vi "UHR-Fleezers Control (host) - 12.7c.vi"() -> ()   [LabVIEW 2012] (continued)
  T19 = typedef "nirio_resource_hc.ctl" = tag
  T20 = typedef "openfpgaref.8.6.ctl" = refnum<k20>
  T21 = enum16{"empty", "write", "read oldest (queue)", "read newest (stack)", "read all"}
  T22 = cluster{"New Image":T2, "New Image":T2, "New Image":T2, "New Image":T2, "New Image":T2}
  T23 = typedef "XDNodeRunTimeDep.lvlib/timing_clust.ctl" = cluster{"Expected End [f-1]":u64, "Actual End [f-1]":u64, "Finished Late? [f-1]":bool, "Expected End [i-1]":u64, "Actual End [i-1]":u64, "Finished Late? [i-1]":bool, "Expected Start [i]":u64, "Actual Start [i]":u64, "Expected Start [f]":u64, "Actual Start [f]":u64, "Source Name":string, "Structure Name":string, "Period":i64, "Deadline":i64, "Offset":i64, "Start":i64, "Priority":i32, "Timeout":i32, "Mode":T24, "Wakeup Reason":T25, "Error":errorcluster, "Source Type":string, "Secondary Source Type":string, "Global End Time":u64, "Global Start Time":u64, "Frame Duration":u64, "Iteration Duration":u64, "Assigned CPU":i32, "I/O Scan Engine Mode":u32}
  T24 = typedef "XDNodeRunTimeDep.lvlib/nitl_modes.ctl" = enum32{"No Change", "Process missed periods, maintain original phase", "Discard missed periods, maintain original phase", "Process missed periods, ignore original phase", "Discard missed periods, ignore original phase"}
  T25 = typedef "XDNodeRunTimeDep.lvlib/wakeup.ctl" = enum32{"Normal", "Aborted", "Asynchronous wakeup", "Timing source error", "Timed loop error", "Timeout"}
  T26 = enum16{"big-endian, network order", "native, host order", "little-endian"}
  T27 = enum16{"open", "replace", "create", "open or create", "replace or create", "replace or create with confirmation"}
  T28 = cluster{"Scan Range AOD (nm) 2":dbl, "Step Size AOD (nm) 2":dbl, "Scan Speed AOD (nm/s) 2":dbl, "Number of scans (AOD) 2":u16, "Label":string}
  T29 = cluster{"[0]":dbl, "[1]":dbl, "[2]":dbl, "[3]":dbl, "[4]":dbl, "[5]":dbl}
  T30 = cluster{"Diameter (mm)":dbl, "Units":dbl, "Volume":dbl, "Rate":dbl}
  T31 = cluster{"Left":i32, "Top":i32, "Width":u32, "Height":u32}
  T32 = cluster{cluster{"Left":i32, "Top":i32, "Width":u32, "Height":u32}}[]
  T33 = enum32{"Status", "Sample Stage", "Syringe Pump", "Trap Control (RF)", "APD Counting", "Fluorescence Laser Control", "Trap AI", "Video", "FPGA"}
  T34 = enum32{"Status", "Sample Stage", "Syringe Pump", "Trap Control (RF)", "APD Counting", "Fluorescence Laser Control", "Trap AI", "Video", "FPGA", "Misc. Configuration"}
  T35 = enum32{"setting", "request", "request control", "info", "statistics", "system settings", "I/O sub system", "HRT control", "camera descriptions", "device specific data", "event sub system settings", "event sub system results", "image memory manager"}
  T36 = typedef "AviRefnum.ctl" = refnum<k1>
  T37 = typedef "imagedata.ctl" = cluster{"image type":i32, "image depth":i32, "image":u8[], "mask":u8[], "colors":u32[], "Rectangle":cluster{"left":i16, "top":i16, "right":i16, "bottom":i16}}
  T38 = enum32{"Normal Display", "Dual Display (APD)", "FFT", "High Res Display"}
  T39 = cluster{"Origin Pixel":cluster{"X":sgl, "Y":sgl}, "Angle Relative to Horizontal (deg)":sgl, "Axis Reference":u32}
  T40 = typedef "Simple Grid Descriptor" = cluster{"X Step":sgl, "Y Step":sgl, "Unit":T41}
  T41 = typedef "Image Unit" = enum32{"Undefined", "Angström", "Micrometer", "Millimeter", "Centimeter", "Meter", "Kilometer", "Microinch", "Inch", "Feet", "Nautical miles", "Standard miles", "Steps"}
  T42 = cluster{"averaging mode":u16, "weighting mode":u16, "number of averages":u32}
  T43 = cluster{"dB On (F)":bool, "unwrap phase (F)":bool, "convert to degree (F)":bool}
  T44 = cluster{string, string, string, string, string, string, string, string}
  T45 = cluster{string, string, string, string, string, string, string, string, string, string, string, string}
  T46 = cluster{string, string, string, string, string, string, string, string, string, string, string, string, string}
  T47 = cluster{string, string, string, string, string, string, string, string, string, string, string, string, string, string}
  T48 = cluster{"BD 1 Frequency 1 (MHz)":dbl, "BD 1 Frequency 2 (MHz)":dbl}
  T49 = cluster{"f0":dbl, "df":dbl, "magnitude":dbl[]}[][]
  T50 = cluster{"Comment (data description)":string, "Channel 1 Buffer":string, "Channel 2 Buffer":string, "Channel 3 Buffer":string, "Title":string, "DNA Construct":string, "Bead diameter":dbl, "Name":string}
diagram:
  w14 = u16 10 items=["1.0"=10, "1.5"=15, "2.0"=20] ("stop bits (10: 1 bit)")
  w80 = u16 20 items=["1.0"=10, "1.5"=15, "2.0"=20] ("stop bits (10: 1 bit)")
  w83 = u16 20 items=["1.0"=10, "1.5"=15, "2.0"=20] ("stop bits (10: 1 bit)")
  w109 = u16 20 items=["1.0"=10, "1.5"=15, "2.0"=20] ("stop bits (10: 1 bit)")
  w20 = T18 2 items=["Grayscale (U8)", "Grayscale (I16)", "Grayscale (SGL)", "Complex (CSG)", "RGB (U32)", "HSL (U32)", "RGB (U64)", "Grayscale (U16)"] ("Image Type")
  w239 = 10.0 ("y")
  w238 = 32767.0 ("y")
  w254 = 6.0  # clock mult.
  w255 = 49152000.0  # TCXO frequ.
  # "Trap X limits"
  # "What are these?"
  # "I don't think you need to do this.\nEverytime you want to adjust phase you always set this anyway.\nSince we removed the separate +/- controls.\n\nHaven't added for added fl lasers.  Should remove this code."
  # "Bottom 1 Harvard"
  # "Top 3 Harvard"
  # "Center Harvard"
  # "Bottom 1 Harvard"
  # "Top 3 Harvard"
  # "Center Harvard"
  n1 = Build Array("DIO count 1 (ticks)", "DIO count 2 (ticks)", "DIO count 3 (ticks)") -> (w160:u16[])
  n2 = xnode "Open FPGA VI Reference"("resource name"=T19 "750kHzDAQ") -> ("FPGA VI Reference Out"=w263:T20, "error out"=w262:errorcluster)  [unwired: 1 in]
  n3 = local read "AO1"() -> (w233:dbl)
  n4 = local read "AO2"() -> (w232:dbl)
  n5 = local read "Scan Increment (MHz)"() -> (w250:dbl)
  n6 = local read "Continuous MCL Scanning"() -> (w220:bool)
  n7 = local read "Fast Scan Dir"() -> (w219:bool)
  n8 = xnode "Invoke Method"("FPGA VI Reference In"=w263, "error in"=w262) -> ("FPGA VI Reference Out"=w1:T20, "error out"=w179:errorcluster)
  n9 = local read "Number of scans (MCL)"() -> (w221:u64)
  n10 = Multiply(x=w233, y=w238) -> (x*y=w235:dbl)
  n11 = Multiply(x=w232, y=w238) -> (x*y=w237:dbl)
  n12 = Divide(x=w235, y=w239) -> (x/y=w234:dbl)
  n13 = Divide(x=w237, y=w239) -> (x/y=w236:dbl)
  n14 = To Word Integer(number=w234) -> (16bit integer=w231:i16)
  n15 = To Word Integer(number=w236) -> (16bit integer=w230:i16)
  n16 = Not(x=w219) -> (.not. x?=w214:bool)
  n17 = local read "Cycles/step (MCL)"() -> (w222:u64)
  n18 = Multiply(x=w250, y=1000.0) -> (x*y=w257:dbl)
  n19 = local read "Scan steps (MCL)"() -> (w223:u64)
  n20 = local read "Desired Scan Incr (V)"() -> (w225:dbl)
  n21 = Scale By Power Of 2(n=48, x=w257) -> (x*2^n=w258:dbl)
  n22 = Unbundle By Name(cluster{"output high":i16, "output low":i16} {"output high"=3000, "output low"=0} ("FB output range 1")) -> ("output high"=w61:i16, "output low"=w60:i16)
  n23 = Multiply(x=w255, y=w254) -> (x*y=w253:dbl)
  n24 = Divide(x=w258, y=w253) -> (x/y=w252:dbl)
  n25 = local read "Setpoints (V)"() -> (w269:cluster{"Set 1":dbl, "Set 2":dbl})
  n26 = To Quad Integer(1:w252) -> (0:w249:i64)
  n27 = Divide(x=40000000.0, y="AI Count (ticks)") -> (x/y=w210:dbl)
  n28 = Multiply(x=w225, y=32767.0) -> (x*y=w227:dbl)
  n29 = local read "Trap Intensity PID Gains"() -> (w264:T9)
  n30 = local read "Next trap write delay (ticks)"() -> (w6:u8)
  n31 = local read "XY phase ext loop method"() -> (w5:bool)
  n32 = local read "Amp switch delay 2"() -> (w4:u8)
  n33 = local read "BD 2 Delay (Ticks) 2"() -> (w3:u8)
  n34 = local read "BD 1 Delay (ticks) 2"() -> (w2:u8)
  n35 = local write "Trap Pos FIFO Timeout"(u16 0 ("Trap Pos FIFO Timeout")) -> ()
  n36 = local read "Number Interlace Sets"() -> (w153:u8)
  n37 = Split 1D Array(array=w160, index=w153) -> (first subarray=w162:u16[])  [unwired: 1 out]
  n38 = Add Array Elements(numeric array=w162) -> (sum=w161:u16)
  n39 = local read "# Samples/channel"() -> (w242:u32)
  n40 = local read "Number of F/B Scans (AOD)"() -> (w243:u16)
  n41 = local read "Not-Interlacing Set"() -> (w152:enum32{"Set 1", "Set 2", "Set 3"})
  n42 = To Unsigned Byte Integer(number=w152) -> (unsigned 8bit integer=w158:u8)
  n43 = Index Array(array=w160, index=w158) -> (element=w159:u16)
  n44 = local read "Feedback On/Off"() -> (w272:cluster{"Set 1":bool, "Set 2":bool})
  n45 = local read "BD 2 Delay (Ticks)"() -> (w7:u8)
  n46 = local read "BD 1 Delay (ticks)"() -> (w8:u8)
  n47 = local read "Scan steps (AOD)"() -> (w248:u64)
  n48 = local read "All FB On/Off"() -> (w273:bool)
  n49 = local read "Cycles/step (AOD)"() -> (w247:u64)
  n50 = local write "AI rate (Hz)"(w210) -> ()
  n51 = Divide(x=w227, y=10.0) -> (x/y=w226:dbl)
  n52 = Multiply(x=w248, y=w247) -> (x*y=w246:u64)
  n53 = Unbundle By Name(w264) -> ("proportional gain (Kc)"=w65:i16, "integral gain (Kc*Ts/Ti)"=w64:i16, "derivative gain (Kc*Td/Ts)"=w63:i16)
  n54 = property on="AI Count (ticks)" class="DigNum (strict)"("Val(Sgnl)"="AI Count (ticks)") -> ()  [unwired: 2 in, 2 out]
  n55 = Multiply(x=3276.7, y=w269) -> (x*y=w268:cluster{"Set 1":dbl, "Set 2":dbl})
  n56 = To Word Integer(number=w226) -> (16bit integer=w224:i16)
  n57 = Multiply(x=w246, y=u64 2) -> (x*y=w244:u64)
  n58 = Divide(x=w210, y="FPGA Ave.") -> (x/y=w211:dbl)
  n59 = To Word Integer(number=w268) -> (16bit integer=w267:cluster{"Set 1":i16, "Set 2":i16})
  n60 = Multiply(x=w244, y=w243) -> (x*y=w241:u64)
  n61 = local read "Sets to FIFO (Traps)"() -> (w69:T15)
  n62 = local write "Ave. Rate (Hz)"(w211) -> ()
  n63 = Divide(x=w241, y=w242) -> (x/y=w240:dbl)
  n64 = Unbundle By Name(w267) -> ("Set 1"=w266:i16, "Set 2"=w265:i16)
  n65 = local read "2D or 1D Scan"() -> (w171:bool)
  n66 = local write "Data points/scans"(w241) -> ()
  n67 = local read "Scan BD"() -> (w259:bool)
  n68 = And(x=w272, y=w273) -> (x .and. y?=w271:cluster{"Set 1":bool, "Set 2":bool})
  n69 = local write "Data points/scan (f/b)"(w244) -> ()
  n70 = Reciprocal(x=w211) -> (1/x=w212:dbl)
  n71 = local read "N Acq Sets (Traps + Fl.)"() -> (w203:i16)
  n72 = local write "N sets should be saved"(w240) -> ()
  n73 = Unbundle By Name(w271) -> ("Set 1"=w275:bool, "Set 2"=w274:bool)
  n74 = local read "Interlace"() -> (w154:bool)
  n75 = Select(t=w161, s=w154, f=w159) -> (s? t:f=w151:u16)
  n76 = local write "Update Count (MCL)"(w151) -> ()
  n77 = local write "Total Counts (ticks)"(w151) -> ()
  n78 = local write "Ave. Period (s)"(w212) -> ()
  n79 = Unbundle By Name(w69) -> ("Set 1"=w68:bool, "Set 2"=w67:bool, "Set 3"=w66:bool)
  n80 = property on="2D or 1D Scan" class="Bool (strict)"("Val(Sgnl)"=w171) -> ()  [unwired: 2 in, 2 out]
  n81 = xnode "Read/Write Control"("FPGA VI Reference In"=w170, "error in"=w179, "ai count"="AI Count (ticks)", "Interlace ON/OFF"=w154, "Number Interlace Cycles"=w153, "Set 1"=w68, "Set 2"=w67, "Set 3"=w66, "FB On/Off Set 1"=w275, "FB On/Off Set 2"=w274, "Interlace Off Parameters"=w152, "FB Setpoint Set 1"=w266, "FB Setpoint Set 2"=w265, "P1"=w65, "I1"=w64, "D1"=w63, "FB1 output high"=w61, "FB1 output low"=w60, "Cycles per step"=w247, "Scan BD"=w259, "Number of scans"=w243, "Scan steps"=w248, "Scan freq.  increment"=w249, "AO1"=w231, "AO2"=w230, "Scan freq.  increment (MCL)"=w224, "Scan steps (MCL)"=w223, "Cycles per step (MCL)"=w222, "Number of scans (MCL)"=w221, "MCL count"=w151, "Cont. Scan (MCL)"=w220, "MCL Scan Axis"=w214, "1D or 2D Scan?"=w171, "N of AI1 Int Acq Sets"=w203, "Amp switch delay"="Amp switch delay", "Swap F1 and F2"="Swap F1 and F2", "APD to FIFO"=FALSE, "DIO count 1 (ticks)"="DIO count 1 (ticks)", "DIO count 2 (ticks)"="DIO count 2 (ticks)", "DIO count 3 (ticks)"="DIO count 3 (ticks)", "BD 1 Delay (ticks)"=w8, "BD 2 Delay (Ticks)"=w7, "Next trap write delay (ticks)"=w6, "XY phase ext loop method"=w5, "Amp switch delay 2"=w4, "BD 2 Delay (Ticks) 2"=w3, "BD 1 Delay (ticks) 2"=w2) -> ("FPGA VI Reference Out"=w25:T20, "error out"=w24:errorcluster)  [unwired: 1 in]
  n82 = local read "Laser interlacing mode"() -> (w150:enum32{"Laser ON", "Laser OFF", "Interlace"})
  n83 = local read "Green Laser ON"() -> (w149:bool)
  n84 = local read "Trap Pos. FB Range"() -> (w59:T12)
  n85 = local read "Trap Pos. FB Gains"() -> (w58:T11)
  n86 = Multiply(x="Green Intensity % (FB OFF)", y=655.35) -> (x*y=w142:dbl)
  n87 = local read "Invert laser interlacing"() -> (w38:bool)
  n88 = local read "Trap Pos. AI1 X Pre-scale"() -> (w97:u16)
  n89 = Multiply(x="Green FB Setpoint (mV)", y=3.2767) -> (x*y=w139:dbl)
  n90 = local read "Trap Pos FB Int Count"() -> (w91:u16)
  n91 = local read "Differential FB?"() -> (w85:bool)
  n92 = local read "Neg. TTrig FPGA"() -> (w87:bool)
  n93 = Multiply(x="Red FB Setpoint (mV)", y=3.2767) -> (x*y=w46:dbl)
  n94 = To Unsigned Word Integer(number=w142) -> (unsigned 16bit integer=w140:u16)
  n95 = Multiply(x="Red Intensity % (FB OFF)", y=655.35) -> (x*y=w42:dbl)
  n96 = To Word Integer(number=w139) -> (16bit integer=w137:i16)
  n97 = Unbundle By Name("Green FB Gains") -> ("proportional gain (Kc)"=w50:i16, "integral gain (Kc*Ts/Ti)"=w49:i16, "derivative gain (Kc*Td/Ts)"=w48:i16)
  n98 = Unbundle By Name("Red FB Gains") -> ("proportional gain (Kc)"=w35:i16, "integral gain (Kc*Ts/Ti)"=w34:i16, "derivative gain (Kc*Td/Ts)"=w33:i16)
  n99 = case shown="False" w149 {
    tunnel: w150 -> [_ w301]
    tunnel: [enum32{"Laser ON", "Laser OFF", "Interlace"}."Laser OFF" ("Green laser mode") w301] -> w37
    frame False {
    }
    frame True {
    }
  }
  n100 = To Word Integer(number=w46) -> (16bit integer=w43:i16)
  n101 = Unbundle By Name(w58) -> ("proportional gain (Kc)"=w54:fxp<+/-,16,8>, "integral gain (Kc*Ts/Ti)"=w53:fxp<+/-,16,8>, "derivative gain (Kc*Td/Ts)"=w52:fxp<+/-,16,8>)
  n102 = To Unsigned Word Integer(number=w42) -> (unsigned 16bit integer=w39:u16)
  n103 = Unbundle By Name(w59) -> ("output high"=w57:fxp<+/-,16,1>, "output low"=w55:fxp<+/-,16,1>)
  n104 = local read "Trap Pos FB Monitor\nT1 or T2"() -> (w102:bool)
  n105 = local read "Trap Pos FB Negate Action"() -> (w101:bool)
  n106 = local read "Trap Pos. FB Offset Factor"() -> (w100:i64)
  n107 = local read "Trap Pos. FB Mult Factor"() -> (w99:i64)
  n108 = xnode "Read/Write Control"("FPGA VI Reference In"=w25, "error in"=w24, "Invert GI 2"=w38, "Operating Mode 2"=w37, "P3"=w50, "I3"=w49, "D3"=w48, "Green FB Setpoint"=w137, "Green FB On/Off"="Green FB On/Off", "Current Out"=w140, "Green int current ON count adj"="Green int current ON count adj", "Operating Mode"=w37, "Invert GI"=w38, "Trap Pos FB Monitor T1 or T2"=w102, "Trap Pos FB Negate Action"=w101, "Trap Pos. FB Offset Factor"=w100, "Trap Pos. FB Mult Factor"=w99, "Force feedback"=FALSE, "AI1 X Scale"=w97, "Trap Pos to FIFO"=TRUE, "Trap Pos FB Int Count"=w91, "TTrig Negate Pos"=w87, "FB Trig Integrate"="FB Trig Integrate", "Diff FB Measurement?"=w85, "Negate Diff?"="Negate Diff?", "P2"=w54, "I2"=w53, "D2"=w52, "FB2 output high"=w57, "FB2 output low"=w55, "Red FB Setpoint"=w43, "RI Current Out"=w39, "Red Laser Operating Mode"=w37, "RI Operating Mode 2"=w37, "Invert RI 2"=w38, "Invert RI"=w38, "P4"=w35, "I4"=w34, "D4"=w33, "Red FB On/Off"="Red FB On/Off") -> ("FPGA VI Reference Out"=w29:T20, "error out"=w31:errorcluster)
  n109 = stacked-sequence {
    tunnel: w31 -> [_ _ _ w312]
    tunnel: [_ _ _ w312] -> w30
    tunnel: w29 -> [_ _ _ w313]
    tunnel: [_ _ _ w313] -> w28
    frame #0 {
      w302 = T21."empty" ("mode")
      # "Clear external fluorescence triggering FIFO"
      # "APD loop counts"
      # "Fluorescence loop counts (rates)"
      n110 = local read "APD Integration Time (s)"() -> (w304:dbl)
      n111 = local read "Interlace ON count"() -> (w305:u16)
      n112 = call "Smart Buffer (DBL) 1.vi"("mode"=w302) -> ()  [unwired: 5 in, 6 out]
      n113 = call "Smart Buffer (DBL) 2.vi"("mode"=w302) -> ()  [unwired: 5 in, 6 out]
      n114 = property on="APD Integration Time (s)" class="DigNum (strict)"("Val(Sgnl)"=w304) -> ()  [unwired: 2 in, 2 out]
      n115 = property on="Interlace ON count" class="DigNum (strict)"("Val(Sgnl)"=w305) -> ()  [unwired: 2 in, 2 out]
      "Number of APDs" <- 3.0 ("Number of APDs")
    }
    frame #1 {
      # "Number of APDs affects\nAPD DMA transfer"
      # "General settings for all lasers:"
      # "And includes all laser\nON/OFF settings"
      # "Fluorescent lasers settings:"
      # "Blue laser settings:"
      n116 = local read "Laser interlacing mode"() -> (w307:enum32{"Laser ON", "Laser OFF", "Interlace"})
      n117 = local read "Invert laser interlacing"() -> (w306:bool)
      n118 = local read "Blue FB On/Off"() -> (w308:bool)
      n119 = property on="Blue FB On/Off" class="Bool (strict)"("Val(Sgnl)"=w308) -> ()  [unwired: 2 in, 2 out]
      n120 = property on="Invert laser interlacing" class="Bool (strict)"("Val(Sgnl)"=w306) -> ()  [unwired: 2 in, 2 out]
      n121 = property on="Laser interlacing mode" class="RadioBtnsControl (strict)"("Val(Sgnl)"=w307) -> ()  [unwired: 2 in, 2 out]
    }
    frame #2 {
      w309 = path "C:/Home/wheeler/Comstock-LabView-Link.udl" ("connection information")
      # "Initialize the database connection"
      n122 = call-poly <vilib>:"DB Tools Open Connection.vi"("connection information"=w309) -> ("connection reference"=w310:T17)  [unwired: 7 in, 1 out]
      "connection reference" <- w310
      n123 = local write "connection reference"(w310) -> ()
      n124 = local write "Database link"(w309) -> ()
    }
    frame #3 {
      n125 = Wait (ms)(milliseconds to wait=u32 1000) -> ()  [unwired: 1 out]
    }
  }
  n126 = local write "Offset (nm)"(0.0 ("Offset (nm)")) -> ()
  n127 = local write "Bead Mean (nm)"(0.0 ("Bead Mean (nm)")) -> ()
  n128 = case shown="\"2axisAOD\"" "1axis AOM vs 2 axis AOD" {
    tunnel: [T16 {"Minimum"=0.0, "Maximum"=40.0, "Increment"=0.1} ("Min Max Inc") T16 {"Minimum"=60.0, "Maximum"=90.0, "Increment"=1.0} ("Min Max Inc")] -> w11
    tunnel: [T16 {"Minimum"=0.0, "Maximum"=45.0, "Increment"=1.0} ("Data Entry Limits") T16 {"Minimum"=0.0, "Maximum"=50.0, "Increment"=1.0} ("Data Entry Limits")] -> w9
    frame "2axisAOD" {
      # "Amp Limits"
      # "Freq Limits"
      n129 = disable-structure shown="Disabled" {
        frame Disabled {
          w319 = 35.0 ("BD 1 Amplitude 1 (%)")
          w320 = 30.0 ("BD 1 Frequency 1 (MHz)")
          n130 = local write "BD 1 Frequency 1 (MHz)"(w320) -> ()
          n131 = local write "BD 1 Frequency 2 (MHz)"(w320) -> ()
          n132 = local write "BD 1 Amplitude 2 (%)"(w319) -> ()
          n133 = local write "BD 1 Amplitude 1 (%)"(w319) -> ()
          n134 = local write "BD 2 Frequency 1 (MHz)"(w320) -> ()
          n135 = local write "BD 2 Amplitude 1 (%)"(w319) -> ()
          n136 = local write "BD 2 Frequency 2 (MHz)"(w320) -> ()
          n137 = local write "BD 2 Amplitude 2 (%)"(w319) -> ()
        }
        frame Enabled {
        }
      }
      n138 = local write "BD 2 Delay (Ticks)"(u8 47 ("BD 2 Delay (Ticks)")) -> ()
      n139 = local write "All FB On/Off"(FALSE ("All FB On/Off")) -> ()
      n140 = local write "Number Interlace Sets"(u8 2 ("Number Interlace Sets")) -> ()
    }
    frame "1axis", Default {
      # "Amp Lmits"
      # "Freq Limits"
    }
  }
  n141 = xnode "Invoke Method"("FPGA VI Reference In"=w28, "error in"=w30, "Requested Depth"="Trap AI FIFO Depth") -> ("FPGA VI Reference Out"=w105:T20, "error out"=w104:errorcluster)  [unwired: 1 out]
  n142 = xnode "Invoke Method"("FPGA VI Reference In"=w105, "error in"=w104, "Requested Depth"="Trap Position FIFO Depth") -> ("FPGA VI Reference Out"=w93:T20, "error out"=w92:errorcluster)  [unwired: 1 out]
  n143 = flat-sequence "Safety limits on RF frequencies and amplitudes (for AOM protection)" {
    tunnel: w1 -> [w327]
    tunnel: [w327] -> w170
    tunnel: [w324] -> w169
    tunnel: [w323] -> w168
    tunnel: [w325] -> w166
    tunnel: [w326] -> w167
    tunnel: w11 -> [w324]
    tunnel: w9 -> [w323]
    frame #0 {
      w326 = T16 {"Minimum"=0.0, "Maximum"=40.0, "Increment"=0.1} ("Min Max Inc")
      w325 = T16 {"Minimum"=0.0, "Maximum"=45.0, "Increment"=1.0} ("Data Entry Limits")
      n144 = property on="BD 2 Frequency 1 (MHz)" class="DigNum (strict)"("Data Range"=w326) -> ()  [unwired: 2 in, 2 out]
      n145 = property on="BD 2 Frequency 3 (MHz)" class="DigNum (strict)"("Data Range"=w326) -> ()  [unwired: 2 in, 2 out]
      n146 = property on="BD 2 Frequency 2 (MHz)" class="DigNum (strict)"("Data Range"=w326) -> ()  [unwired: 2 in, 2 out]
      n147 = property on="BD 1 Frequency 1 (MHz)" class="DigNum (strict)"("Data Range"=w324) -> ()  [unwired: 2 in, 2 out]
      n148 = property on="BD 1 Frequency 2 (MHz)" class="DigNum (strict)"("Data Range"=w324) -> ()  [unwired: 2 in, 2 out]
      n149 = property on="BD 1 Frequency 3 (MHz)" class="DigNum (strict)"("Data Range"=w324) -> ()  [unwired: 2 in, 2 out]
      n150 = property on="BD 2 Amplitude 1 (%)" class="DigNum (strict)"("Data Range"=w325) -> ()  [unwired: 2 in, 2 out]
      n151 = property on="BD 2 Amplitude 2 (%)" class="DigNum (strict)"("Data Range"=w325) -> ()  [unwired: 2 in, 2 out]
      n152 = property on="BD 2 Amplitude 3 (%)" class="DigNum (strict)"("Data Range"=w325) -> ()  [unwired: 2 in, 2 out]
      n153 = property on="BD 1 Amplitude 3 (%)" class="DigNum (strict)"("Data Range"=w323) -> ()  [unwired: 2 in, 2 out]
      n154 = property on="BD 1 Amplitude 2 (%)" class="DigNum (strict)"("Data Range"=w323) -> ()  [unwired: 2 in, 2 out]
      n155 = property on="BD 1 Amplitude 1 (%)" class="DigNum (strict)"("Data Range"=w323) -> ()  [unwired: 2 in, 2 out]
      "X RF Frequency Limits (MHz)" <- w324
      "X RF Amplitude Limits (%)" <- w323
      "Y RF Amplitude Limits (%)" <- w325
      "Y RF Frequency Limits (MHz)" <- w326
    }
  }
  n156 = xnode "Invoke Method"("FPGA VI Reference In"=w93, "error in"=w92) -> ("FPGA VI Reference Out"=w178:T20, "error out"=w177:errorcluster)  [unwired: 1 in]
  n157 = flat-sequence "Initial FPGA Loop Relative Phase Adjustment" {
    tunnel: "Initial Phase Adjustment (AI1)" -> [w342]
    tunnel: "Initial Phase Adjustment (GI)" -> [w341]
    tunnel: w178 -> [w340]
    tunnel: w177 -> [w339]
    tunnel: "Initial Phase Adj. (MCL)" -> [w338]
    tunnel: [w343] -> w187
    tunnel: [w337] -> w183
    tunnel: "Initial Phase Adjustment (APD Acq)" -> [w336]
    tunnel: "Initial Phase Adjustment (APD 1 Gate)" -> [w335]
    tunnel: "Initial Phase Adjustment (Green FB)" -> [w334]
    tunnel: "Initial Phase Adjustment (GI) 2" -> [w333]
    tunnel: "Initial Phase Adjustment (APD 2 Gate)" -> [w332]
    tunnel: "Initial Phase Adjustment (RI)" -> [w331]
    tunnel: "Initial Phase Adjustment (BI DO)" -> [w330]
    tunnel: "Initial Phase Adjustment (BI AO)" -> [w329]
    tunnel: "Initial Phase Adjustment (APD 3 Gate)" -> [w328]
    tunnel: w187 -> [w345]
    tunnel: [w346] -> w184
    tunnel: w183 -> [w346]
    tunnel: [w345] -> w182
    tunnel: w184 -> [w349]
    tunnel: w182 -> [w348]
    tunnel: [w351] -> w181
    tunnel: [w350] -> w180
    tunnel: [w353] -> w185
    tunnel: [w354] -> w186
    tunnel: w181 -> [w354]
    tunnel: w180 -> [w353]
    frame #0 {
      n158 = xnode "Read/Write Control"("FPGA VI Reference In"=w340, "error in"=w339, "Phase count adjustment"=w342, "Phase count adjustment (GI)"=w341, "Phase count adjustment (MCL)"=w338, "Phase Count Adjustment (APD Acq)"=w336, "Phase count adjustment (APD 1 Gate)"=w335, "Phase count adjustment (APD 2 Gate)"=w332, "Phase count adjustment (Green FB)"=w334, "Phase count adjustment (GI) 2"=w333, "Phase count adjustment (RI)"=w331, "Phase count adjustment (BI AO)"=w329, "Phase count adjustment (BI D)"=w330, "Phase count adjustment (APD 3 Gate)"=w328) -> ("FPGA VI Reference Out"=w337:T20, "error out"=w343:errorcluster)
    }
    frame #1 {
      n159 = Wait (ms)(milliseconds to wait=u32 100) -> ()  [unwired: 1 out]
    }
    frame #2 {
      w347 = TRUE
      n160 = xnode "Read/Write Control"("FPGA VI Reference In"=w349, "error in"=w348, "+ phase"=w347, "+ phase (GI)"=w347, "+ phase (MCL)"=w347, "+ phase (APD Acq)"=w347, "+ phase (APD 1 Gate)"=w347, "+ phase (APD 2 Gate)"=w347, "+ phase (Green FB)"=w347, "+ phase (GI) 2"=w347, "+ phase (RI)"=w347, "+ phase (BI AO)"=w347, "+ phase (BI D)"=w347, "+ phase (APD 3 Gate)"=w347) -> ("FPGA VI Reference Out"=w350:T20, "error out"=w351:errorcluster)
    }
    frame #3 {
      n161 = Wait (ms)(milliseconds to wait=u32 100) -> ()  [unwired: 1 out]
    }
  }
  n162 = local read "Phase adj. (Green FB)"() -> (w163:i16)
  n163 = local read "Phase adj. (GI) 2"() -> (w143:i16)
  n164 = local read "Phase adjust (MCL)"() -> (w215:i16)
  n165 = local read "Phase adj. (AI1)"() -> (w217:i16)
  n166 = local read "Phase adj. (GI)"() -> (w216:i16)
  n167 = xnode "Read/Write Control"("FPGA VI Reference In"=w185, "error in"=w186, "Phase count adjustment"=w217, "Phase count adjustment (GI)"=w216, "Phase count adjustment (MCL)"=w215, "Phase Count Adjustment (APD Acq)"="Phase Adj. (APD Acq)", "Phase count adjustment (APD 1 Gate)"="Phase Adj. (APD 1 Gate)", "Phase count adjustment (APD 2 Gate)"="Phase Adj. (APD 2 Gate)", "Phase count adjustment (Green FB)"=w163, "Phase count adjustment (GI) 2"=w143) -> ("FPGA VI Reference Out"=w129:T20, "error out"=w192:errorcluster)
  n168 = call "Initialize RF boards - interlace 3.vi"("error in"=w192, "FPGA VI Reference In"=w129) -> ("error out"=w190:errorcluster, "FPGA VI Reference Out"=w191:T20)
  n169 = call "set RF board frequency - interlace.vi"("Board 2 Frequency Limits"=w167, "Board 1 Frequency Limits"=w169, "error in"=w190, "FPGA VI Reference In"=w191, "Board 2 Frequency 3 (MHz)"="BD 2 Frequency 3 (MHz)", "Board 1 Frequency 3 (MHz)"="BD 1 Frequency 3 (MHz)", "Board 2 Frequency 2 (MHz)"="BD 2 Frequency 2 (MHz)", "Board 2 Frequency 1 (MHz)"="BD 2 Frequency 1 (MHz)", "Board 1 Frequency 2 (MHz)"="BD 1 Frequency 2 (MHz)", "Board 1 Frequency 1  (MHz)"="BD 1 Frequency 1 (MHz)") -> ("error out"=w290:errorcluster, "FPGA VI Reference Out"=w291:T20)
  n170 = call "set RF board amplitude - interlace.vi"("Board 2 Amplitude Limits"=w166, "Board 1 Amplitude Limits"=w168, "error in"=w290, "FPGA VI Reference In"=w291, "Board 2 Amplitude 3 (%)"="BD 2 Amplitude 3 (%)", "Board 1 Amplitude 3 (%)"="BD 1 Amplitude 3 (%)", "Board 2 Amplitude 2 (%)"="BD 2 Amplitude 2 (%)", "Board 2 Amplitude 1 (%)"="BD 2 Amplitude 1 (%)", "Board 1 Amplitude 2 (%)"="BD 1 Amplitude 2 (%)", "Board 1 Amplitude 1 (%)"="BD 1 Amplitude 1 (%)") -> ("error out"=w278:errorcluster, "FPGA VI Reference Out"=w279:T20)
  n171 = flat-sequence {
    tunnel: w279 -> [w364]
    tunnel: w278 -> [w363]
    tunnel: [w362] -> w283
    tunnel: [w361] -> w282
    tunnel: [w368] -> w281
    tunnel: w283 -> [w368]
    tunnel: [w367] -> w280
    tunnel: w282 -> [w367]
    tunnel: w281 -> [w377]
    tunnel: w280 -> [w376]
    tunnel: [w375] -> w23
    tunnel: [w374] -> w94
    frame #0 {
      w355 = FALSE ("Retract Pump 3")
      n172 = local read "Trap 1 (ON/OFF)"() -> (w356:bool)
      n173 = xnode "Read/Write Control"("FPGA VI Reference In"=w364, "error in"=w363, "Direct RF Box  Communication"=FALSE) -> ("FPGA VI Reference Out"=w362:T20, "error out"=w361:errorcluster)
      n174 = local write "Saving..."(FALSE ("Saving Data")) -> ()
      n175 = local write "Stop All"(FALSE ("Stop All")) -> ()
      n176 = local write "Retract Pump 1"(w355) -> ()
      n177 = local write "Retract Pump 3"(w355) -> ()
      n178 = local write "Index"(1.0 ("Index")) -> ()
      n179 = property on="Trap 1 ON" class="Bool (strict)"("Value"=w356) -> ()  [unwired: 2 in, 2 out]
      "Manipulating Trap" <- FALSE ("Manipulating Trap")
    }
    frame #1 {
      n180 = local read "Trap 2 (ON/OFF)"() -> (w366:bool)
      n181 = Wait (ms)(milliseconds to wait=u32 10) -> ()  [unwired: 1 out]
      n182 = property on="Trap 2 ON" class="Bool (strict)"("Val(Sgnl)"=w366) -> ()  [unwired: 2 in, 2 out]
    }
    frame #2 {
      n183 = local read "Scan Range (nm)"() -> (w370:dbl)
      n184 = xnode "Read/Write Control"("FPGA VI Reference In"=w377, "error in"=w376, "FPGA Controls  RF Box"=TRUE ("Direct RF Box  Communication")) -> ("FPGA VI Reference Out"=w375:T20, "error out"=w374:errorcluster)
      n185 = call "Update messages.vi"("Message to add"="UHR-Fleezers ready.", "Old message string"="") -> ("New message string"=w373:string)
      n186 = local write "Messages"(w373) -> ()
      n187 = property on="Scan Range (nm)" class="DigNum (strict)"("Val(Sgnl)"=w370) -> ()  [unwired: 2 in, 2 out]
    }
  }
  n188 = Subtract(x="BD 1 Frequency 1 (MHz)", y="BD 1 Frequency 2 (MHz)") -> (x-y=w202:dbl)
  n189 = Subtract(x="BD 2 Frequency 1 (MHz)", y="BD 2 Frequency 2 (MHz)") -> (x-y=w201:dbl)
  n190 = Square(x=w201) -> (x^2=w199:dbl)
  n191 = Square(x=w202) -> (x^2=w200:dbl)
  n192 = Add(x=w200, y=w199) -> (x+y=w198:dbl)
  n193 = Square Root(x=w198) -> (sqrt(x)=w197:dbl)
  n194 = local write "Trap Delta (MHz)"(w197) -> ()
  n195 = call-poly "VISA Configure Serial Port"("VISA resource name"="VISA resource name", "baud rate (9600)"=u32 115200, "stop bits (10: 1 bit)"=w14) -> ("VISA resource name out"=w13:refnum<visa-resource-name>, "error out"=w12:errorcluster)  [unwired: 4 in, 7 out]
  n196 = call-poly "VISA Configure Serial Port"("VISA resource name"="Bottom  1 Harvard Syringe Pump Serial Port", "baud rate (9600)"=u32 115200, "stop bits (10: 1 bit)"=w80) -> ("VISA resource name out"=w76:refnum<visa-resource-name>, "error out"=w75:errorcluster)  [unwired: 4 in, 7 out]
  n197 = call-poly "VISA Configure Serial Port"("VISA resource name"="Top 3 Harvard Syringe Pump Serial Port", "baud rate (9600)"=u32 115200, "stop bits (10: 1 bit)"=w83) -> ("VISA resource name out"=w78:refnum<visa-resource-name>, "error out"=w77:errorcluster)  [unwired: 4 in, 7 out]
  n198 = call-poly "VISA Configure Serial Port"("VISA resource name"="Sample Chamber Stage Serial Port") -> ("VISA resource name out"=w124:refnum<visa-resource-name>, "error out"=w125:errorcluster)  [unwired: 5 in, 8 out]
  "Stage Control Serial Error" <- w125
  n199 = local write "Blue Error Out"(w12) -> ()
  n200 = call-poly "VISA Configure Serial Port"("VISA resource name"="Center Harvard Syringe Pump Serial Port", "baud rate (9600)"=u32 115200, "stop bits (10: 1 bit)"=w109) -> ("VISA resource name out"=w106:refnum<visa-resource-name>, "error out"=w107:errorcluster)  [unwired: 4 in, 7 out]
  n201 = call "IMAQ Create"("Image Name"="APD 1 Image", "Image Type"=w20) -> ("New Image"=w115:T2)  [unwired: 3 in, 1 out]
  n202 = call "IMAQ Create"("Image Name"="APD 2 Image", "Image Type"=w20) -> ("New Image"=w114:T2)  [unwired: 3 in, 1 out]
  n203 = call "IMAQ Create"("Image Name"="APD 3 Image", "Image Type"=w20) -> ("New Image"=w19:T2)  [unwired: 3 in, 1 out]
  n204 = call "IMAQ Create"("Image Name"="Det. X Image", "Image Type"=w20) -> ("New Image"=w113:T2)  [unwired: 3 in, 1 out]
  n205 = call "IMAQ Create"("Image Name"="Det. Y Image", "Image Type"=w20) -> ("New Image"=w112:T2)  [unwired: 3 in, 1 out]
  n206 = Bundle("New Image"=w115, "New Image"=w114, "New Image"=w19, "New Image"=w113, "New Image"=w112) -> (w111:T22)  [unwired: 1 in]
  n207 = node-c288(3 ("Processor")) -> (w131:T23)  [unwired: 3 out]
  n208 = node-c288(2 ("Processor")) -> (w133:T23)  [unwired: 3 out]
  n209 = node-c288() -> (w18:T23)  [unwired: 4 out]
  n210 = node-c288() -> (w135:T23)  [unwired: 4 out]
  n211 = node-c288() -> (w120:T23)  [unwired: 4 in]
  n212 = while "Duncan's play event loop" {
    stop <- w380 stop-if-true
    n213 = Create User Event(user event datatype=TRUE ("Boolean")) -> (user event=w381:refnum<user-event>)  [unwired: 1 in, 1 out]
    n214 = Create User Event(user event datatype=TRUE ("Boolean")) -> (user event=w388:refnum<user-event>)  [unwired: 1 in, 1 out]
    n215 = global write "Global for fluorescence simulation mean (30 samples), (power series).vi" "Red Signal"(w381) -> ()
    n216 = global write "Global for fluorescence simulation mean (30 samples), (power series).vi" "Green Signal"(w388) -> ()
    n217 = register-events(w388, w381) -> (reference out=w387:refnum<event-registration>)  [unwired: 2 in, 1 out]
    n218 = event shown="[1] \"Get Fluorophore\": Value Change" {
      selector: w387 -> [_ _ _ _]
      dyn-events: _ -> [_ _ _ _]
      timeout: 100 -> [_ _ _ _]
      event Timeout {
        n219 = event-data() -> ()  [unwired: 1 in, 2 out]
      }
      event "Get Fluorophore": Value Change {
        n220 = event-data() -> ("OldVal"=w390:bool)  [unwired: 1 in, 4 out]
        n221 = case shown="True" w390 {
          selector: w390 -> [_ w391]
          frame False {
          }
          frame True {
            n222 = property on="Move to Position 3" class="Bool"("Val(Sgnl)"=w391) -> ()  [unwired: 2 in, 2 out]
            n223 = case shown="1" "Numeric" {
              frame 0, Default {
              }
              frame 1 {
                n224 = property on="Green Laser ON" class="Bool (strict)"("Val(Sgnl)"=TRUE ("Value (Signaling)")) -> ()  [unwired: 2 in, 2 out]
              }
              frame 2 {
                n225 = property on="Red Laser ON" class="Bool (strict)"("Val(Sgnl)"=TRUE) -> ()  [unwired: 2 in, 2 out]
              }
            }
          }
        }
      }
      event User Event {
        n226 = event-data() -> ("Boolean"=w395:bool)  [unwired: 1 in, 3 out]
        "Green Fluorophore" <- w395
        n227 = property on="Get Fluorophore" class="Bool (strict)"("Val(Sgnl)"=w395) -> ()  [unwired: 2 in, 2 out]
      }
      event User Event {
        n228 = event-data() -> ("Boolean"=w396:bool)  [unwired: 1 in, 3 out]
        "Red Fluorophore" <- w396
        n229 = property on="Get Fluorophore" class="Bool (strict)"("Val(Sgnl)"=w396) -> ()  [unwired: 2 in, 2 out]
      }
    }
    n230 = property on="Get Fluorophore" class="Bool (strict)"("Val(Sgnl)"="Get Fluorophore") -> ()  [unwired: 2 in, 2 out]
    n231 = Wait (ms)(milliseconds to wait=u32 100) -> ()  [unwired: 1 out]
    n232 = local read "Stop All"() -> (w379:bool)
    n233 = Or(x=w379, y="stop") -> (x .or. y?=w380:bool)
  }
  n234 = timed-loop "Oscillate Trap/AOM (fishing, conjugate plane alignment)" {
    tunnel: w1 -> [w398]
    tunnel: [w397] -> w136
    timing: w131 -> [_]
    timing-out: [_] -> w130
    stop <- w397 stop-if-true
    n235 = node-c288() -> ()  [unwired: 2 out]
    n236 = event shown="[0] \"Oscillate Set 1\", \"Fish for Tether\": Value Change" {
      selector: _ -> [_ _ _]
      dyn-events: _ -> [_ _ _]
      timeout: _ -> [_ _ _]
      tunnel: w398 -> [w405 _ _]
      tunnel: [FALSE ("Stop All") _ w1003] -> w397
      event "Oscillate Set 1", "Fish for Tether": Value Change {
        n237 = event-data() -> ()  [unwired: 6 out]
        n238 = local read "Oscillate Set 1"() -> (w404:bool)
        n239 = Or(x=w404, y="Fish for Tether") -> (x .or. y?=w402:bool)
        n240 = case shown="True" w402 {
          tunnel: w405 -> [_ w408]
          tunnel: "Fish for Tether" -> [_ w407]
          frame False {
          }
          frame True {
            n241 = case shown="True" w407 {
              selector: w407 -> [w411 w417]
              tunnel: [w411 w417] -> w406
              frame False {
              }
              frame True {
                n242 = local write "Scan axis 2"(TRUE) -> ()
                n243 = local write "Tether"(FALSE ("Tether")) -> ()
                n244 = local read "Flow ON during cal?"() -> (w412:bool)
                n245 = property on="Trap Delta (MHz)" class="DigNum (strict)"("Val(Sgnl)"="Furthest Delta (MHz)") -> ()  [unwired: 2 in, 2 out]
                n246 = Or(x="Flow ON during \nfishing?", y=w412) -> (x .or. y?=w413:bool)
                n247 = Wait (ms)(milliseconds to wait=u32 500) -> ()  [unwired: 1 out]
                n248 = property on="Sample Channel\nFlow" class="Bool (strict)"("Val(Sgnl)"=w413) -> ()  [unwired: 2 in, 2 out]
              }
            }
            n249 = node-c288() -> (w410:T23)  [unwired: 1 in, 3 out]
            n250 = timed-loop "Oscillate AOD" {
              timing: w410 -> [_]
              timing-out: [_] -> w409
              tunnel: w408 -> [w427]
              tunnel: w406 -> [w420]
              i -> [w429]
              stop <- w426 stop-if-true
              n251 = node-c288() -> (w428:i64)  [unwired: 1 out]
              n252 = flat-sequence {
                tunnel: w429 -> [w456]
                tunnel: w428 -> [w455]
                tunnel: w427 -> [w437]
                tunnel: w420 -> [w439]
                tunnel: [w439] -> w425
                tunnel: [w438] -> w424
                tunnel: [w436] -> w423
                tunnel: [w433] -> w421
                tunnel: w425 -> [w501]
                tunnel: w424 -> [w499]
                tunnel: w423 -> [w498]
                tunnel: [w497] -> w422
                tunnel: w421 -> [w496]
                tunnel: [w573] -> w426
                tunnel: w422 -> [w572]
                frame #0 {
                  # "w (rad/s)"
                  # "t (s)"
                  n253 = Divide(x=w455, y=i64 1000) -> (x/y=w430:dbl)
                  n254 = local read "BD 1 Frequency 2 (MHz)"() -> (w432:dbl)
                  n255 = Multiply(x="Osc. freq. (Hz)", y=6.283185307179586) -> (x*y=w453:dbl)
                  n256 = Multiply(x=w430, y=w456) -> (x*y=w452:dbl)
                  n257 = Multiply(x=w453, y=w452) -> (x*y=w435:dbl)
                  n258 = local read "BD 1 Frequency 1 (MHz)"() -> (w441:dbl)
                  n259 = case shown="True" w439 {
                    tunnel: w435 -> [w462 w479]
                    tunnel: w441 -> [_ w487]
                    tunnel: w432 -> [_ w488]
                    tunnel: [w459 w483] -> w431
                    tunnel: [FALSE w464] -> w436
                    tunnel: [0.0 w475] -> w433
                    frame False {
                      n260 = Sine(x=w462) -> (sin(x)=w460:dbl)
                      n261 = Multiply(x=w460, y="Osc. amp. (MHz)") -> (x*y=w459:dbl)
                    }
                    frame True {
                      # "trap position goes from 0 to 1 (0 is when it is furthest away, 1 is when closest)\nso we want to test for tether only when farther away, or x < 1"
                      # "quit if taking too long"
                      # "oscillate the trap"
                      # "Test for tether"
                      n262 = local read "Vec Mean of T1 T2"() -> (w463:dbl[])
                      "Trigger Signal" <- w463
                      n263 = Cosine(x=w479) -> (cos(x)=w491:dbl)
                      n264 = Subtract(x=w488, y=w487) -> (x-y=w486:dbl)
                      n265 = Decrement(x=w491) -> (x-1=w490:dbl)
                      n266 = Subtract(x=w486, y="Closest Delta (MHz)") -> (x-y=w484:dbl)
                      n267 = Divide(x=w490, y=-2.0) -> (x/y=w474:dbl)
                      n268 = Greater?(x=w463, y="Stop F (pN)") -> (0:w481:bool[])
                      n269 = Multiply(x=w474, y=w484) -> (x*y=w483:dbl)
                      n270 = Less?(x=w474, y="Fish mask thresh") -> (x < y?=w473:bool)
                      n271 = Boolean To (0,1)(Boolean=w473) -> (0, 1=w471:i16)
                      n272 = Multiply(x=w471, y=w463) -> (x*y=w470:dbl[])
                      n273 = Divide(x=w479, y=6.283185307179586) -> (x/y=w478:dbl)
                      n274 = Round Toward +Infinity(x=w478) -> (ceil(x): smallest int >= x=w475:dbl)
                      "Attempts" <- w475
                      n275 = Greater?(x=w470, y="Stop F (pN) (mask)") -> (0:w468:bool[])
                      n276 = Or Array Elements(Boolean array=w481) -> (logical OR=w466:bool)
                      n277 = Or Array Elements(Boolean array=w468) -> (logical OR=w465:bool)
                      n278 = Greater?(x=w475, y="Attempt Limit") -> (0:w477:bool)
                      n279 = case shown="True" w477 {
                        frame False {
                        }
                        frame True {
                          n280 = local write "Fish for Tether"(FALSE ("Fish for Tether")) -> ()
                          n281 = call <vilib>:"Beep.vi"() -> ()  [unwired: 3 in, 9 out]
                          n282 = local read "Messages"() -> (w493:string)
                          n283 = call "Update messages.vi"("Message to add"="Tether fishing timeout." ("Messages"), "Old message string"=w493) -> ("New message string"=→"Messages":string)
                        }
                      }
                      n284 = Select(t=w466, s="Normal (on) or masked test (off)", f=w465) -> (s? t:f=w464:bool)
                    }
                  }
                  n285 = local read "BD 2 Frequency 1 (MHz)"() -> (w440:dbl)
                  n286 = Select(t=w441, s="Scan axis 2", f=w440) -> (s? t:f=w444:dbl)
                  n287 = Add(x=w431, y=w444) -> (x+y=w438:dbl)
                  n288 = Select(t=w438, s="Scan axis 2", f=w441) -> (s? t:f=w447:dbl)
                  n289 = Select(t=w440, s="Scan axis 2", f=w438) -> (s? t:f=w446:dbl)
                  n290 = local read "BD 2 Frequency 2 (MHz)"() -> (w449:dbl)
                  n291 = local read "BD 2 Frequency 3 (MHz)"() -> (w448:dbl)
                  n292 = local read "Y RF Frequency Limits (MHz)"() -> (w442:T16)
                  n293 = local read "X RF Frequency Limits (MHz)"() -> (w443:T16)
                  n294 = local read "BD 1 Frequency 3 (MHz)"() -> (w450:dbl)
                  n295 = call "set RF board frequency - interlace.vi"("Board 2 Frequency Limits"=w442, "Board 1 Frequency Limits"=w443, "FPGA VI Reference In"=w437, "Board 2 Frequency 3 (MHz)"=w448, "Board 1 Frequency 3 (MHz)"=w450, "Board 2 Frequency 2 (MHz)"=w449, "Board 2 Frequency 1 (MHz)"=w446, "Board 1 Frequency 2 (MHz)"=w432, "Board 1 Frequency 1  (MHz)"=w447) -> ()  [unwired: 1 in, 2 out]
                }
                frame #1 {
                  n296 = And(x=w501, y=w498) -> (x .and. y?=w500:bool)
                  n297 = case "Only if were fishing and now formed tether" shown="True" w500 {
                    tunnel: w499 -> [w503 w518]
                    tunnel: [w502 w517] -> w497
                    tunnel: w496 -> [_ w513]
                    frame False {
                      n298 = local read "Fish for Tether"() -> (w502:bool)
                      n299 = case shown="False" w502 {
                        tunnel: w503 -> [w504 _]
                        frame False {
                          n300 = property on="BD 1 Frequency 1 (MHz)" class="DigNum (strict)"("Val(Sgnl)"=w504) -> ()  [unwired: 2 in, 2 out]
                        }
                        frame True {
                        }
                      }
                    }
                    frame True {
                      w517 = FALSE ("Fish for Tether")
                      n301 = call <vilib>:"Beep.vi"() -> ()  [unwired: 3 in, 9 out]
                      n302 = Number To Decimal String(number=w513, width (-)=i16 1) -> (decimal integer string=w511:string)
                      n303 = Concatenate Strings("Formed tether in ", w511, " attempt(s)." ("string")) -> (w508:string)
                      n304 = local read "Messages"() -> (w515:string)
                      n305 = local write "Fish for Tether"(w517) -> ()
                      n306 = call "Update messages.vi"("Message to add"=w508, "Old message string"=w515) -> ("New message string"=w514:string)
                      n307 = local write "Messages"(w514) -> ()
                      n308 = Get Date/Time In Seconds() -> (seconds since 1Jan1904=→"Time tether formed":timestamp)
                      n309 = local read "Flow ON during cal?"() -> (w505:bool)
                      n310 = property on="Sample Channel\nFlow" class="Bool (strict)"("Val(Sgnl)"=w505) -> (error out=w506:errorcluster)  [unwired: 2 in, 1 out]
                      n311 = case shown="\"2\", \"3\", \"4\", \"5\", \"6\"" "Then..." {
                        selector: "Then..." -> [_ w521]
                        tunnel: w518 -> [w520 _]
                        tunnel: w506 -> [_ _]
                        frame "1", Default {
                          n312 = property on="BD 1 Frequency 1 (MHz)" class="DigNum (strict)"("Val(Sgnl)"=w520) -> ()  [unwired: 2 in, 2 out]
                        }
                        frame "2", "3", "4", "5", "6" {
                          n313 = flat-sequence {
                            tunnel: w521 -> [w523]
                            frame #0 {
                              n314 = property on="Trap Delta (MHz)" class="DigNum (strict)"("Val(Sgnl)"="Move to Delta 1 (MHz)") -> ()  [unwired: 2 in, 2 out]
                            }
                            frame #1 {
                              n315 = case shown="\"5\", \"6\"" w523 {
                                selector: w523 -> [w526 w536 _]
                                frame "3", "4" {
                                n316 = flat-sequence {
                                tunnel: w526 -> [w527]
                                tunnel: [w527] -> w524
                                tunnel: [w529] -> w525
                                tunnel: w524 -> [w529]
                                tunnel: w525 -> [w533]
                                frame #0 {
                                n317 = property on="Green Laser ON" class="Bool (strict)"("Val(Sgnl)"=TRUE ("Value (Signaling)")) -> ()  [unwired: 2 in, 2 out]
                                }
                                frame #1 {
                                n318 = Multiply(x="Wait Before Save (s)", y=u32 1000 ("x")) -> (x*y=w531:u32)
                                n319 = Wait (ms)(milliseconds to wait=w531) -> ()  [unwired: 1 out]
                                }
                                frame #2 {
                                n320 = property on="Start Saving" class="Bool (strict)"("Value"=TRUE ("Start Saving")) -> ()  [unwired: 2 in, 2 out]
                                n321 = case shown="\"4\"" w533 {
                                frame Default {
                                }
                                frame "4" {
                                n322 = property on="Fl. Triggered..." class="Bool (strict)"("Val(Sgnl)"=TRUE ("Value (Signaling)")) -> ()  [unwired: 2 in, 2 out]
                                }
                                }
                                }
                                }
                                }
                                frame "5", "6" {
                                n323 = stacked-sequence {
                                tunnel: w536 -> [_ _ _ _ _ _ w548]
                                frame #0 {
                                n324 = Replace Array Subset(array=u32[] [0] ("Index Values"), new element="Raster Set Upon Tether", index=0) -> (w537:u32[])
                                n325 = property on="Saved AOD Raster Scan Parameter Sets" class="Arr (strict)"("Index Values"=w537) -> ()  [unwired: 2 in, 2 out]
                                }
                                frame #1 {
                                n326 = Wait (ms)(milliseconds to wait=u32 500) -> ()  [unwired: 1 out]
                                }
                                frame #2 {
                                n327 = property on="Load parameters" class="Bool (strict)"("Val(Sgnl)"=TRUE ("Value (Signaling)")) -> ()  [unwired: 2 in, 2 out]
                                n328 = case shown="True" "Green ON During Raster" {
                                frame False {
                                }
                                frame True {
                                n329 = property on="Green Laser ON" class="Bool (strict)"("Val(Sgnl)"=TRUE ("Value (Signaling)")) -> ()  [unwired: 2 in, 2 out]
                                }
                                }
                                }
                                frame #3 {
                                n330 = Wait (ms)(milliseconds to wait=u32 500) -> ()  [unwired: 1 out]
                                }
                                frame #4 {
                                n331 = property on="Trap Raster Scan" class="Bool (strict)"("Val(Sgnl)"=TRUE ("Value (Signaling)")) -> ()  [unwired: 2 in, 2 out]
                                }
                                frame #5 {
                                n332 = Wait (ms)(milliseconds to wait=u32 2000) -> ()  [unwired: 1 out]
                                }
                                frame #6 {
                                n333 = flat-sequence {
                                tunnel: w548 -> [w555]
                                frame #0 {
                                n334 = while {
                                stop <- w551 stop-if-true
                                n335 = local read "Raster Scanning..."() -> (w550:bool)
                                n336 = local read "Saving..."() -> (w553:bool)
                                n337 = Wait (ms)(milliseconds to wait=u32 100) -> ()  [unwired: 1 out]
                                n338 = Not(x=w553) -> (.not. x?=w552:bool)
                                n339 = Not(x=w550) -> (.not. x?=w549:bool)
                                n340 = And(x=w552, y=w549) -> (x .and. y?=w551:bool)
                                }
                                }
                                frame #1 {
                                n341 = local read "Tether"() -> (w556:bool)
                                n342 = case shown="True" w556 {
                                tunnel: w555 -> [_ w558]
                                frame False {
                                n343 = property on="Fish for Tether" class="Bool (strict)"("Val(Sgnl)"="Fish again after \nraster break?") -> ()  [unwired: 2 in, 2 out]
                                }
                                frame True {
                                n344 = stacked-sequence {
                                tunnel: w558 -> [_ w562 _ _]
                                frame #0 {
                                n345 = property on="Trap Delta (MHz)" class="DigNum (strict)"("Val(Sgnl)"="Move to Delta 2 (MHz)") -> ()  [unwired: 2 in, 2 out]
                                n346 = case shown="True" "Flow ON after\ntether testing?" {
                                frame False {
                                }
                                frame True {
                                n347 = property on="Sample Channel\nFlow" class="Bool (strict)"("Val(Sgnl)"=TRUE ("Value (Signaling)")) -> ()  [unwired: 2 in, 2 out]
                                }
                                }
                                }
                                frame #1 {
                                n348 = flat-sequence {
                                tunnel: w562 -> [w564]
                                frame #0 {
                                n349 = Wait (ms)(milliseconds to wait=u32 500) -> ()  [unwired: 1 out]
                                }
                                frame #1 {
                                n350 = case shown="\"6\"" w564 {
                                frame Default {
                                }
                                frame "6" {
                                n351 = property on="Green Laser ON" class="Bool (strict)"("Val(Sgnl)"=TRUE ("Green Laser ON/Interlacing")) -> ()  [unwired: 2 in, 2 out]
                                }
                                }
                                }
                                frame #2 {
                                n352 = Wait (ms)(milliseconds to wait=u32 500) -> ()  [unwired: 1 out]
                                }
                                frame #3 {
                                n353 = local write "Start Saving"("Save at end (5, 6)") -> ()
                                }
                                }
                                }
                                frame #2 {
                                n354 = local read "Bead Sep. Int. Time (s)"() -> (w570:dbl)
                                n355 = Multiply(x=w570, y=1000.0) -> (x*y=w569:dbl)
                                n356 = Wait (ms)(milliseconds to wait=w569) -> ()  [unwired: 1 out]
                                }
                                frame #3 {
                                n357 = property on="Remove Offset" class="Bool (strict)"("Val(Sgnl)"=TRUE ("Value (Signaling)")) -> ()  [unwired: 2 in, 2 out]
                                }
                                }
                                }
                                }
                                }
                                }
                                }
                                }
                                }
                                frame "2", Default {
                                }
                              }
                            }
                          }
                        }
                      }
                      "Tether" <- "Tether Alarm?"
                    }
                  }
                }
                frame #2 {
                  n358 = local read "Oscillate Set 1"() -> (w577:bool)